vi "UHR-Fleezers Control (host) - 12.3.vi"() -> ()   [LabVIEW 2012] (continued)
                                }
                                frame #3 {
                                n359 = for {
                                N: 4 -> [_]
                                n360 = flat-sequence {
                                frame #0 {
                                n361 = Wait (ms)(milliseconds to wait=u32 500) -> ()  [unwired: 1 out]
                                }
                                frame #1 {
                                n362 = local read "Action (%)"() -> (w633:dbl)
                                n363 = Absolute Value(x=w633) -> (abs(x)=w632:dbl)
                                n364 = Greater?(x=w632, y=70.0) -> (0:w630:bool)
                                n365 = property on="Remove Action Offset" class="Bool (strict)"("Val(Sgnl)"=w630) -> ()  [unwired: 2 in, 2 out]
                                }
                                }
                                }
                                }
                                frame #4 {
                                n366 = Wait (ms)(milliseconds to wait=u32 500) -> ()  [unwired: 1 out]
                                }
                                frame #5 {
                                n367 = local read "Mean"() -> (w641:dbl)
                                n368 = Greater?(x=w641, y=11.0) -> (0:w635:bool)
                                n369 = Not(x=w635) -> (.not. x?=w636:bool)
                                n370 = And(x=w636, y="Shift confocal") -> (x .and. y?=w638:bool)
                                n371 = And(x=w635, y="Shift confocal") -> (x .and. y?=w639:bool)
                                n372 = case shown="True" w639 {
                                frame False {
                                }
                                frame True {
                                n373 = local read "Confocal Y 2 (V)"() -> (w645:dbl)
                                n374 = local read "Confocal X 2 (V)"() -> (w644:dbl)
                                n375 = property on="AO1" class="Slide (strict)"("Val(Sgnl)"=w645) -> ()  [unwired: 2 in, 2 out]
                                n376 = property on="AO2" class="Slide (strict)"("Val(Sgnl)"=w644) -> ()  [unwired: 2 in, 2 out]
                                }
                                }
                                n377 = case shown="True" w638 {
                                frame False {
                                }
                                frame True {
                                n378 = local read "Confocal Y 1 (V)"() -> (w643:dbl)
                                n379 = local read "Confocal X 1 (V)"() -> (w642:dbl)
                                n380 = property on="AO1" class="Slide (strict)"("Val(Sgnl)"=w643) -> ()  [unwired: 2 in, 2 out]
                                n381 = property on="AO2" class="Slide (strict)"("Val(Sgnl)"=w642) -> ()  [unwired: 2 in, 2 out]
                                }
                                }
                                }
                                frame #6 {
                                n382 = Wait (ms)(milliseconds to wait=u32 1500) -> ()  [unwired: 1 out]
                                }
                                frame #7 {
                                n383 = property on="Rem fb disp offset" class="Bool (strict)"("Val(Sgnl)"=TRUE ("Value (Signaling)")) -> ()  [unwired: 2 in, 2 out]
                                }
                                }
                                }
                                frame True {
                                n384 = flat-sequence {
                                tunnel: w648 -> [w649]
                                frame #0 {
                                n385 = property on="Trap Delta (MHz)" class="DigNum (strict)"("Val(Sgnl)"=w649) -> ()  [unwired: 2 in, 2 out]
                                }
                                frame #1 {
                                n386 = Wait (ms)(milliseconds to wait=u32 500) -> ()  [unwired: 1 out]
                                }
                                frame #2 {
                                n387 = local read "Shift confocal"() -> (w655:bool)
                                n388 = local read "Mean"() -> (w657:dbl)
                                n389 = Greater?(x=w657, y=11.0) -> (0:w654:bool)
                                n390 = Not(x=w654) -> (.not. x?=w653:bool)
                                n391 = And(x=w653, y=w655) -> (x .and. y?=w651:bool)
                                n392 = And(x=w654, y=w655) -> (x .and. y?=w652:bool)
                                n393 = case shown="True" w652 {
                                frame False {
                                }
                                frame True {
                                n394 = local read "Confocal Y 2 (V)"() -> (w661:dbl)
                                n395 = local read "Confocal X 2 (V)"() -> (w660:dbl)
                                n396 = property on="AO2" class="Slide (strict)"("Val(Sgnl)"=w660) -> ()  [unwired: 2 in, 2 out]
                                n397 = property on="AO1" class="Slide (strict)"("Val(Sgnl)"=w661) -> ()  [unwired: 2 in, 2 out]
                                }
                                }
                                n398 = case shown="True" w651 {
                                frame False {
                                }
                                frame True {
                                n399 = local read "Confocal X 1 (V)"() -> (w658:dbl)
                                n400 = local read "Confocal Y 1 (V)"() -> (w659:dbl)
                                n401 = property on="AO2" class="Slide (strict)"("Val(Sgnl)"=w658) -> ()  [unwired: 2 in, 2 out]
                                n402 = property on="AO1" class="Slide (strict)"("Val(Sgnl)"=w659) -> ()  [unwired: 2 in, 2 out]
                                }
                                }
                                }
                                }
                                }
                                }
                                }
                                }
                                }
                                frame "Image" {
                                n403 = property on="Confocal Image" class="Bool (strict)"("Val(Sgnl)"=TRUE ("Value (Signaling)")) -> ()  [unwired: 2 in, 2 out]
                                }
                              }
                              n404 = local write "Fl. High"(FALSE ("Fl. High")) -> ()
                              n405 = local read "Time (s)"() -> (w595:dbl)
                            }
                            frame #1 {
                              n406 = case shown="True" "Auto F Reset" {
                                tunnel: w667 -> [_ w672]
                                tunnel: w666 -> [_ w671]
                                tunnel: w665 -> [_ w670]
                                tunnel: w664 -> [_ w669]
                                frame False {
                                }
                                frame True {
                                n407 = node-c288() -> (w674:T21)  [unwired: 4 in]
                                n408 = timed-loop {
                                timing: w674 -> [_]
                                timing-out: [_] -> w673
                                tunnel: w672 -> [w679]
                                tunnel: w671 -> [w678]
                                tunnel: w670 -> [w677]
                                tunnel: w669 -> [w676]
                                stop <- w675 stop-if-true
                                n409 = node-c288() -> ()  [unwired: 1 in, 1 out]
                                n410 = local read "Fl. Delta Thresh. (kHz)"() -> (w688:dbl)
                                n411 = local read "APD to Watch"() -> (w689:bool)
                                n412 = local read "Delta Fl. 1"() -> (w690:dbl)
                                n413 = local read "Delta Fl. 2"() -> (w691:dbl)
                                n414 = local read "Fl. Triggered..."() -> (w682:bool)
                                n415 = local read "Stop All"() -> (w683:bool)
                                n416 = local read "Reset Force"() -> (w681:bool)
                                n417 = Multiply(x=w688, y=1000.0) -> (x*y=w686:dbl)
                                n418 = Select(t=w690, s=w689, f=w691) -> (s? t:f=w685:dbl)
                                n419 = Not(x=w682) -> (.not. x?=w680:bool)
                                n420 = Greater?(x=w685, y=w686) -> (0:w684:bool)
                                n421 = Compound Arithmetic op=OR(w684, w683, w680, w681) -> (w675:bool)
                                n422 = case shown="True" w675 {
                                tunnel: w679 -> [_ w695]
                                tunnel: w678 -> [_ w699]
                                tunnel: w677 -> [_ w698]
                                tunnel: w676 -> [_ w697]
                                frame False {
                                }
                                frame True {
                                n423 = case shown="\"Yank\"" w699 {
                                tunnel: w698 -> [_ w709]
                                tunnel: w697 -> [_ w707]
                                frame "Image", Default {
                                }
                                frame "Yank" {
                                n424 = flat-sequence {
                                tunnel: [w712] -> w710
                                tunnel: w709 -> [w712]
                                tunnel: [w711] -> w708
                                tunnel: w707 -> [w711]
                                tunnel: w710 -> [w718]
                                tunnel: w708 -> [w716]
                                frame #0 {
                                n425 = local read "Yank Delay (s)"() -> (w715:dbl)
                                n426 = Multiply(x=w715, y=1000.0) -> (x*y=w713:dbl)
                                n427 = Wait (ms)(milliseconds to wait=w713) -> ()  [unwired: 1 out]
                                }
                                frame #1 {
                                n428 = local read "Yank to which?"() -> (w717:bool)
                                n429 = case shown="False" w717 {
                                tunnel: w718 -> [_ w746]
                                tunnel: w716 -> [w719 _]
                                frame False {
                                n430 = flat-sequence {
                                tunnel: w719 -> [w720]
                                frame #0 {
                                n431 = property on="Trap Pos FB SP" class="DigNum (strict)"("Val(Sgnl)"=w720) -> ()  [unwired: 2 in, 2 out]
                                }
                                frame #1 {
                                n432 = Wait (ms)(milliseconds to wait=u32 700) -> ()  [unwired: 1 out]
                                }
                                frame #2 {
                                n433 = local read "Action (%)"() -> (w725:dbl)
                                n434 = Absolute Value(x=w725) -> (abs(x)=w724:dbl)
                                n435 = Greater?(x=w724, y=70.0) -> (0:w722:bool)
                                n436 = property on="Remove Action Offset" class="Bool (strict)"("Val(Sgnl)"=w722) -> ()  [unwired: 2 in, 2 out]
                                }
                                frame #3 {
                                n437 = for {
                                N: 4 -> [_]
                                n438 = flat-sequence {
                                frame #0 {
                                n439 = Wait (ms)(milliseconds to wait=u32 500) -> ()  [unwired: 1 out]
                                }
                                frame #1 {
                                n440 = local read "Action (%)"() -> (w731:dbl)
                                n441 = Absolute Value(x=w731) -> (abs(x)=w730:dbl)
                                n442 = Greater?(x=w730, y=70.0) -> (0:w728:bool)
                                n443 = property on="Remove Action Offset" class="Bool (strict)"("Val(Sgnl)"=w728) -> ()  [unwired: 2 in, 2 out]
                                }
                                }
                                }
                                }
                                frame #4 {
                                n444 = Wait (ms)(milliseconds to wait=u32 500) -> ()  [unwired: 1 out]
                                }
                                frame #5 {
                                n445 = local read "Shift confocal"() -> (w736:bool)
                                n446 = local read "Mean"() -> (w739:dbl)
                                n447 = Greater?(x=w739, y=11.0) -> (0:w735:bool)
                                n448 = Not(x=w735) -> (.not. x?=w734:bool)
                                n449 = And(x=w735, y=w736) -> (x .and. y?=w737:bool)
                                n450 = And(x=w734, y=w736) -> (x .and. y?=w733:bool)
                                n451 = case shown="True" w737 {
                                frame False {
                                }
                                frame True {
                                n452 = local read "Confocal X 2 (V)"() -> (w742:dbl)
                                n453 = local read "Confocal Y 2 (V)"() -> (w743:dbl)
                                n454 = property on="AO2" class="Slide (strict)"("Val(Sgnl)"=w742) -> ()  [unwired: 2 in, 2 out]
                                n455 = property on="AO1" class="Slide (strict)"("Val(Sgnl)"=w743) -> ()  [unwired: 2 in, 2 out]
                                }
                                }
                                n456 = case shown="True" w733 {
                                frame False {
                                }
                                frame True {
                                n457 = local read "Confocal Y 1 (V)"() -> (w741:dbl)
                                n458 = local read "Confocal X 1 (V)"() -> (w740:dbl)
                                n459 = property on="AO1" class="Slide (strict)"("Val(Sgnl)"=w741) -> ()  [unwired: 2 in, 2 out]
                                n460 = property on="AO2" class="Slide (strict)"("Val(Sgnl)"=w740) -> ()  [unwired: 2 in, 2 out]
                                }
                                }
                                }
                                frame #6 {
                                n461 = Wait (ms)(milliseconds to wait=u32 1500) -> ()  [unwired: 1 out]
                                }
                                frame #7 {
                                n462 = property on="Rem fb disp offset" class="Bool (strict)"("Val(Sgnl)"=TRUE ("Value (Signaling)")) -> ()  [unwired: 2 in, 2 out]
                                }
                                }
                                }
                                frame True {
                                n463 = flat-sequence {
                                tunnel: w746 -> [w747]
                                frame #0 {
                                n464 = property on="Trap Delta (MHz)" class="DigNum (strict)"("Val(Sgnl)"=w747) -> ()  [unwired: 2 in, 2 out]
                                }
                                frame #1 {
                                n465 = Wait (ms)(milliseconds to wait=u32 500) -> ()  [unwired: 1 out]
                                }
                                frame #2 {
                                n466 = local read "Shift confocal"() -> (w753:bool)
                                n467 = local read "Mean"() -> (w754:dbl)
                                n468 = Greater?(x=w754, y=11.0) -> (0:w752:bool)
                                n469 = And(x=w752, y=w753) -> (x .and. y?=w750:bool)
                                n470 = Not(x=w752) -> (.not. x?=w751:bool)
                                n471 = And(x=w751, y=w753) -> (x .and. y?=w749:bool)
                                n472 = case shown="True" w750 {
                                frame False {
                                }
                                frame True {
                                n473 = local read "Confocal Y 2 (V)"() -> (w759:dbl)
                                n474 = local read "Confocal X 2 (V)"() -> (w758:dbl)
                                n475 = property on="AO1" class="Slide (strict)"("Val(Sgnl)"=w759) -> ()  [unwired: 2 in, 2 out]
                                n476 = property on="AO2" class="Slide (strict)"("Val(Sgnl)"=w758) -> ()  [unwired: 2 in, 2 out]
                                }
                                }
                                n477 = case shown="True" w749 {
                                frame False {
                                }
                                frame True {
                                n478 = local read "Confocal Y 1 (V)"() -> (w757:dbl)
                                n479 = local read "Confocal X 1 (V)"() -> (w756:dbl)
                                n480 = property on="AO2" class="Slide (strict)"("Val(Sgnl)"=w756) -> ()  [unwired: 2 in, 2 out]
                                n481 = property on="AO1" class="Slide (strict)"("Val(Sgnl)"=w757) -> ()  [unwired: 2 in, 2 out]
                                }
                                }
                                }
                                }
                                }
                                }
                                }
                                }
                                }
                                }
                                n482 = local read "Time (s)"() -> (w694:dbl)
                                n483 = Subtract(x=w695, y=w694) -> (x-y=w706:dbl)
                                n484 = Number To Decimal String(number=w706, width (-)=i16 0) -> (decimal integer string=w704:string)
                                n485 = Concatenate Strings(w704, " s fluorescence event") -> (w701:string)
                                n486 = local read "Messages"() -> (w702:string)
                                n487 = local write "Duration (s)"(w706) -> ()
                                n488 = call "Update messages.vi"("Message to add"=w701, "Old message string"=w702) -> ("New message string"=w700:string)
                                n489 = local write "Messages"(w700) -> ()
                                n490 = call <vilib>:"Beep.vi"() -> ()  [unwired: 12 in]
                                n491 = local write "Reset Force"(FALSE ("Force Reset")) -> ()
                                n492 = local write "Fl. High"(TRUE ("Fl. High")) -> ()
                                n493 = local write "Waiting"(TRUE ("Waiting")) -> ()
                                }
                                }
                                n494 = node-c288() -> ()  [unwired: 1 in, 1 out]
                                }
                                n495 = node-c288(w673) -> ()  [unwired: 1 out]
                                }
                              }
                            }
                          }
                          n496 = local read "Trap Delta (MHz)"() -> (w585:dbl)
                          n497 = local read "Trap Pos FB SP"() -> (w583:fxp<+/-,16,1>)
                        }
                      }
                    }
                    frame True {
                      n498 = flat-sequence {
                        tunnel: w770 -> [w780]
                        tunnel: [w780] -> w774
                        tunnel: w773 -> [w779]
                        tunnel: [w779] -> w772
                        tunnel: [w778] -> w771
                        tunnel: w769 -> [w777]
                        tunnel: [w776] -> w768
                        tunnel: w765 -> [w775]
                        tunnel: [w775] -> w764
                        tunnel: w774 -> [w850]
                        tunnel: w772 -> [w849]
                        tunnel: w771 -> [w848]
                        tunnel: w768 -> [w847]
                        tunnel: w764 -> [w846]
                        tunnel: [w847] -> w767
                        frame #0 {
                          n499 = call <vilib>:"Beep.vi"() -> ()  [unwired: 3 in, 9 out]
                          n500 = local write "Waiting"(FALSE ("Waiting")) -> ()
                          n501 = Increment(x=w777) -> (x+1=w776:u8)
                          n502 = case shown="\"Yank\"" w779 {
                            tunnel: w776 -> [_ _ w786]
                            frame "Image" {
                              n503 = property on="Confocal Image" class="Bool (strict)"("Val(Sgnl)"=TRUE ("Value (Signaling)")) -> ()  [unwired: 2 in, 2 out]
                            }
                            frame "Alarm", Default {
                            }
                            frame "Yank" {
                              n504 = flat-sequence {
                                tunnel: w786 -> [w789]
                                tunnel: [w788] -> w785
                                tunnel: ["N Array El"] -> w784
                                tunnel: w785 -> [w803]
                                tunnel: w784 -> [w799]
                                frame #0 {
                                n505 = Multiply(x="Yank Delay (s)", y=1000.0) -> (x*y=w792:dbl)
                                n506 = Quotient & Remainder(x=w789, y="N Array El") -> (x-y*floor(x/y)=w788:u8)  [unwired: 1 out]
                                n507 = Wait (ms)(milliseconds to wait=w792) -> ()  [unwired: 1 out]
                                }
                                frame #1 {
                                n508 = Random Number (0-1)() -> (number: 0 to 1=w800:dbl)
                                n509 = Multiply(x=w799, y=w800) -> (x*y=w798:dbl)
                                n510 = Round Toward -Infinity(1:w798) -> (0:w797:dbl)
                                n511 = Select(t=w797, s="Random Choice", f=w803) -> (s? t:f=w801:dbl)
                                n512 = Select(t="Yank to Trap Delta (MHz)", s="Yank to which?", f="Yank to SP") -> (s? t:f=w794:dbl[])
                                n513 = Index Array(array=w794, index=w801) -> (element=w804:dbl)
                                n514 = case shown="False" "Yank to which?" {
                                tunnel: w804 -> [w805 w831]
                                frame False {
                                n515 = flat-sequence {
                                tunnel: w805 -> [w806]
                                frame #0 {
                                n516 = property on="Trap Pos FB SP" class="DigNum (strict)"("Val(Sgnl)"=w806) -> ()  [unwired: 2 in, 2 out]
                                }
                                frame #1 {
                                n517 = Wait (ms)(milliseconds to wait=u32 700) -> ()  [unwired: 1 out]
                                }
                                frame #2 {
                                n518 = local read "Action (%)"() -> (w811:dbl)
                                n519 = Absolute Value(x=w811) -> (abs(x)=w810:dbl)
                                n520 = Greater?(x=w810, y=70.0) -> (0:w808:bool)
                                n521 = property on="Remove Action Offset" class="Bool (strict)"("Val(Sgnl)"=w808) -> ()  [unwired: 2 in, 2 out]
                                }
                                frame #3 {
                                n522 = for {
                                N: 4 -> [_]
                                n523 = flat-sequence {
                                frame #0 {
                                n524 = Wait (ms)(milliseconds to wait=u32 500) -> ()  [unwired: 1 out]
                                }
                                frame #1 {
                                n525 = local read "Action (%)"() -> (w817:dbl)
                                n526 = Absolute Value(x=w817) -> (abs(x)=w816:dbl)
                                n527 = Greater?(x=w816, y=70.0) -> (0:w814:bool)
                                n528 = property on="Remove Action Offset" class="Bool (strict)"("Val(Sgnl)"=w814) -> ()  [unwired: 2 in, 2 out]
                                }
                                }
                                }
                                }
                                frame #4 {
                                n529 = local read "Shift confocal"() -> (w821:bool)
                                n530 = local read "Mean"() -> (w824:dbl)
                                n531 = Greater?(x=w824, y=11.0) -> (0:w820:bool)
                                n532 = Not(x=w820) -> (.not. x?=w819:bool)
                                n533 = And(x=w819, y=w821) -> (x .and. y?=w818:bool)
                                n534 = And(x=w820, y=w821) -> (x .and. y?=w822:bool)
                                n535 = case shown="True" w822 {
                                frame False {
                                }
                                frame True {
                                n536 = local read "Confocal X 2 (V)"() -> (w827:dbl)
                                n537 = local read "Confocal Y 2 (V)"() -> (w828:dbl)
                                n538 = property on="AO2" class="Slide (strict)"("Val(Sgnl)"=w827) -> ()  [unwired: 2 in, 2 out]
                                n539 = property on="AO1" class="Slide (strict)"("Val(Sgnl)"=w828) -> ()  [unwired: 2 in, 2 out]
                                }
                                }
                                n540 = case shown="True" w818 {
                                frame False {
                                }
                                frame True {
                                n541 = local read "Confocal X 1 (V)"() -> (w825:dbl)
                                n542 = local read "Confocal Y 1 (V)"() -> (w826:dbl)
                                n543 = property on="AO1" class="Slide (strict)"("Val(Sgnl)"=w826) -> ()  [unwired: 2 in, 2 out]
                                n544 = property on="AO2" class="Slide (strict)"("Val(Sgnl)"=w825) -> ()  [unwired: 2 in, 2 out]
                                }
                                }
                                }
                                frame #5 {
                                n545 = Wait (ms)(milliseconds to wait=u32 1500) -> ()  [unwired: 1 out]
                                }
                                frame #6 {
                                n546 = property on="Rem fb disp offset" class="Bool (strict)"("Val(Sgnl)"=TRUE ("Value (Signaling)")) -> ()  [unwired: 2 in, 2 out]
                                }
                                }
                                }
                                frame True {
                                n547 = flat-sequence {
                                tunnel: w831 -> [w832]
                                frame #0 {
                                n548 = property on="Trap Delta (MHz)" class="DigNum (strict)"("Val(Sgnl)"=w832) -> ()  [unwired: 2 in, 2 out]
                                }
                                frame #1 {
                                n549 = Wait (ms)(milliseconds to wait=u32 500) -> ()  [unwired: 1 out]
                                }
                                frame #2 {
                                n550 = local read "Shift confocal"() -> (w836:bool)
                                n551 = local read "Mean"() -> (w834:dbl)
                                n552 = Greater?(x=w834, y=11.0) -> (0:w837:bool)
                                n553 = Not(x=w837) -> (.not. x?=w838:bool)
                                n554 = And(x=w838, y=w836) -> (x .and. y?=w840:bool)
                                n555 = And(x=w837, y=w836) -> (x .and. y?=w839:bool)
                                n556 = case shown="True" w839 {
                                frame False {
                                }
                                frame True {
                                n557 = local read "Confocal Y 2 (V)"() -> (w844:dbl)
                                n558 = local read "Confocal X 2 (V)"() -> (w843:dbl)
                                n559 = property on="AO1" class="Slide (strict)"("Val(Sgnl)"=w844) -> ()  [unwired: 2 in, 2 out]
                                n560 = property on="AO2" class="Slide (strict)"("Val(Sgnl)"=w843) -> ()  [unwired: 2 in, 2 out]
                                }
                                }
                                n561 = case shown="True" w840 {
                                frame False {
                                }
                                frame True {
                                n562 = local read "Confocal X 1 (V)"() -> (w841:dbl)
                                n563 = local read "Confocal Y 1 (V)"() -> (w842:dbl)
                                n564 = property on="AO2" class="Slide (strict)"("Val(Sgnl)"=w841) -> ()  [unwired: 2 in, 2 out]
                                n565 = property on="AO1" class="Slide (strict)"("Val(Sgnl)"=w842) -> ()  [unwired: 2 in, 2 out]
                                }
                                }
                                }
                                }
                                }
                                }
                                }
                              }
                            }
                          }
                          n566 = local read "Time (s)"() -> (w778:dbl)
                          "Fl. High" <- TRUE ("Yanking")
                        }
                        frame #1 {
                          n567 = local read "Auto F Reset"() -> (w845:bool)
                          n568 = case shown="True" w845 {
                            tunnel: w850 -> [_ w854]
                            tunnel: w849 -> [_ w853]
                            tunnel: w848 -> [_ w852]
                            tunnel: w846 -> [_ w851]
                            frame False {
                            }
                            frame True {
                              n569 = node-c288() -> (w856:T21)  [unwired: 4 out]
                              n570 = timed-loop {
                                timing: w856 -> [_]
                                timing-out: [_] -> w855
                                tunnel: w854 -> [w874]
                                tunnel: w853 -> [w873]
                                tunnel: w852 -> [w872]
                                tunnel: w851 -> [w871]
                                stop <- w857 stop-if-true
                                n571 = node-c288() -> ()  [unwired: 2 out]
                                n572 = local read "Fl. Delta Thresh. (kHz)"() -> (w865:dbl)
                                n573 = local read "Fl. Triggered..."() -> (w870:bool)
                                n574 = local read "Delta Fl. 1"() -> (w861:dbl)
                                n575 = local read "Delta Fl. 2"() -> (w859:dbl)
                                n576 = local read "Stop All"() -> (w868:bool)
                                n577 = local read "APD to Watch"() -> (w860:bool)
                                n578 = Select(t=w861, s=w860, f=w859) -> (s? t:f=w858:dbl)
                                n579 = Not(x=w870) -> (.not. x?=w869:bool)
                                n580 = Multiply(x=w865, y=1000.0) -> (x*y=w864:dbl)
                                n581 = Negate(x=w864) -> (-x=w863:dbl)
                                n582 = Less?(x=w858, y=w863) -> (x < y?=w867:bool)
                                n583 = Compound Arithmetic op=OR(w867, w868, w869, "Reset Force") -> (w857:bool)
                                n584 = case shown="True" w857 {
                                tunnel: w874 -> [_ w889]
                                tunnel: w873 -> [_ w888]
                                tunnel: w872 -> [_ w878]
                                tunnel: w871 -> [_ w880]
                                frame False {
                                }
                                frame True {
                                n585 = local read "Time (s)"() -> (w879:dbl)
                                n586 = case shown="\"Yank\"" w888 {
                                tunnel: w889 -> [_ w892]
                                tunnel: w880 -> [_ w890]
                                frame "Image", Default {
                                }
                                frame "Yank" {
                                n587 = flat-sequence {
                                tunnel: [w898] -> w893
                                tunnel: w892 -> [w898]
                                tunnel: [w894] -> w891
                                tunnel: w890 -> [w894]
                                tunnel: w893 -> [w901]
                                tunnel: w891 -> [w899]
                                frame #0 {
                                n588 = local read "Yank Delay (s)"() -> (w897:dbl)
                                n589 = Multiply(x=w897, y=1000.0) -> (x*y=w895:dbl)
                                n590 = Wait (ms)(milliseconds to wait=w895) -> ()  [unwired: 1 out]
                                }
                                frame #1 {
                                n591 = local read "Yank to which?"() -> (w900:bool)
                                n592 = case shown="False" w900 {
                                tunnel: w901 -> [_ w928]
                                tunnel: w899 -> [w902 _]
                                frame False {
                                n593 = flat-sequence {
                                tunnel: w902 -> [w903]
                                frame #0 {
                                n594 = property on="Trap Pos FB SP" class="DigNum (strict)"("Val(Sgnl)"=w903) -> ()  [unwired: 2 in, 2 out]
                                }
                                frame #1 {
                                n595 = Wait (ms)(milliseconds to wait=u32 700) -> ()  [unwired: 1 out]
                                }
                                frame #2 {
                                n596 = local read "Action (%)"() -> (w908:dbl)
                                n597 = Absolute Value(x=w908) -> (abs(x)=w907:dbl)
                                n598 = Greater?(x=w907, y=70.0) -> (0:w905:bool)
                                n599 = property on="Remove Action Offset" class="Bool (strict)"("Val(Sgnl)"=w905) -> ()  [unwired: 2 in, 2 out]
                                }
                                frame #3 {
                                n600 = for {
                                N: 4 -> [_]
                                n601 = flat-sequence {
                                frame #0 {
                                n602 = Wait (ms)(milliseconds to wait=u32 500) -> ()  [unwired: 1 out]
                                }
                                frame #1 {
                                n603 = local read "Action (%)"() -> (w914:dbl)
                                n604 = Absolute Value(x=w914) -> (abs(x)=w913:dbl)
                                n605 = Greater?(x=w913, y=70.0) -> (0:w911:bool)
                                n606 = property on="Remove Action Offset" class="Bool (strict)"("Val(Sgnl)"=w911) -> ()  [unwired: 2 in, 2 out]
                                }
                                }
                                }
                                }
                                frame #4 {
                                n607 = local read "Shift confocal"() -> (w919:bool)
                                n608 = local read "Mean"() -> (w921:dbl)
                                n609 = Greater?(x=w921, y=11.0) -> (0:w918:bool)
                                n610 = Not(x=w918) -> (.not. x?=w917:bool)
                                n611 = And(x=w918, y=w919) -> (x .and. y?=w916:bool)
                                n612 = And(x=w917, y=w919) -> (x .and. y?=w915:bool)
                                n613 = case shown="True" w916 {
                                frame False {
                                }
                                frame True {
                                n614 = local read "Confocal Y 2 (V)"() -> (w925:dbl)
                                n615 = local read "Confocal X 2 (V)"() -> (w924:dbl)
                                n616 = property on="AO2" class="Slide (strict)"("Val(Sgnl)"=w924) -> ()  [unwired: 2 in, 2 out]
                                n617 = property on="AO1" class="Slide (strict)"("Val(Sgnl)"=w925) -> ()  [unwired: 2 in, 2 out]
                                }
                                }
                                n618 = case shown="True" w915 {
                                frame False {
                                }
                                frame True {
                                n619 = local read "Confocal X 1 (V)"() -> (w922:dbl)
                                n620 = local read "Confocal Y 1 (V)"() -> (w923:dbl)
                                n621 = property on="AO1" class="Slide (strict)"("Val(Sgnl)"=w923) -> ()  [unwired: 2 in, 2 out]
                                n622 = property on="AO2" class="Slide (strict)"("Val(Sgnl)"=w922) -> ()  [unwired: 2 in, 2 out]
                                }
                                }
                                }
                                frame #5 {
                                n623 = Wait (ms)(milliseconds to wait=u32 1500) -> ()  [unwired: 1 out]
                                }
                                frame #6 {
                                n624 = property on="Rem fb disp offset" class="Bool (strict)"("Val(Sgnl)"=TRUE ("Value (Signaling)")) -> ()  [unwired: 2 in, 2 out]
                                }
                                }
                                }
                                frame True {
                                n625 = flat-sequence {
                                tunnel: w928 -> [w929]
                                frame #0 {
                                n626 = property on="Trap Delta (MHz)" class="DigNum (strict)"("Val(Sgnl)"=w929) -> ()  [unwired: 2 in, 2 out]
                                }
                                frame #1 {
                                n627 = Wait (ms)(milliseconds to wait=u32 500) -> ()  [unwired: 1 out]
                                }
                                frame #2 {
                                n628 = local read "Shift confocal"() -> (w935:bool)
                                n629 = local read "Mean"() -> (w937:dbl)
                                n630 = Greater?(x=w937, y=11.0) -> (0:w934:bool)
                                n631 = Not(x=w934) -> (.not. x?=w933:bool)
                                n632 = And(x=w934, y=w935) -> (x .and. y?=w932:bool)
                                n633 = And(x=w933, y=w935) -> (x .and. y?=w931:bool)
                                n634 = case shown="True" w932 {
                                frame False {
                                }
                                frame True {
                                n635 = local read "Confocal Y 2 (V)"() -> (w941:dbl)
                                n636 = local read "Confocal X 2 (V)"() -> (w940:dbl)
                                n637 = property on="AO2" class="Slide (strict)"("Val(Sgnl)"=w940) -> ()  [unwired: 2 in, 2 out]
                                n638 = property on="AO1" class="Slide (strict)"("Val(Sgnl)"=w941) -> ()  [unwired: 2 in, 2 out]
                                }
                                }
                                n639 = case shown="True" w931 {
                                frame False {
                                }
                                frame True {
                                n640 = local read "Confocal Y 1 (V)"() -> (w939:dbl)
                                n641 = local read "Confocal X 1 (V)"() -> (w938:dbl)
                                n642 = property on="AO2" class="Slide (strict)"("Val(Sgnl)"=w938) -> ()  [unwired: 2 in, 2 out]
                                n643 = property on="AO1" class="Slide (strict)"("Val(Sgnl)"=w939) -> ()  [unwired: 2 in, 2 out]
                                }
                                }
                                }
                                }
                                }
                                }
                                }
                                }
                                }
                                }
                                n644 = local read "Messages"() -> (w887:string)
                                n645 = Subtract(x=w879, y=w878) -> (x-y=w885:dbl)
                                "Duration (s)" <- w885
                                n646 = Number To Decimal String(number=w885, width (-)=i16 0) -> (decimal integer string=w883:string)
                                n647 = Concatenate Strings(w883, " s fluorescence event." ("string")) -> (w881:string)
                                n648 = call "Update messages.vi"("Message to add"=w881, "Old message string"=w887) -> ("New message string"=w886:string)
                                n649 = local write "Reset Force"(FALSE ("Reset Force")) -> ()
                                n650 = local write "Waiting"(TRUE ("Waiting")) -> ()
                                n651 = local write "Messages"(w886) -> ()
                                n652 = local write "Fl. High"(FALSE ("Fl. High")) -> ()
                                n653 = call <vilib>:"Beep.vi"() -> ()  [unwired: 3 in, 9 out]
                                }
                                }
                                n654 = node-c288() -> ()  [unwired: 2 out]
                              }
                              n655 = node-c288(w855) -> ()  [unwired: 1 out]
                            }
                          }
                        }
                      }
                      n656 = local read "Trap Delta (MHz)"() -> (w770:dbl)
                      n657 = local read "Trap Pos FB SP"() -> (w765:fxp<+/-,16,1>)
                    }
                  }
                }
                frame #1 {
                  n658 = local read "Stop All"() -> (w951:bool)
                  n659 = local read "Fl. Triggered..."() -> (w949:bool)
                  n660 = Not(x=w949) -> (.not. x?=w950:bool)
                  n661 = Or(x=w950, y=w951) -> (x .or. y?=w948:bool)
                }
              }
              n662 = case shown="True" w542 {
                frame False {
                }
                frame True {
                  n663 = local read "Confocal Y 1 (V)"() -> (w552:dbl)
                  n664 = local read "Confocal X 1 (V)"() -> (w551:dbl)
                  n665 = property on="AO2" class="Slide (strict)"("Val(Sgnl)"=w551) -> ()  [unwired: 2 in, 2 out]
                  n666 = property on="AO1" class="Slide (strict)"("Val(Sgnl)"=w552) -> ()  [unwired: 2 in, 2 out]
                }
              }
              n667 = case shown="True" w542 {
                frame False {
                }
                frame True {
                  w550 = FALSE ("Fl. High")
                  n668 = local write "Waiting"(w550) -> ()
                  n669 = local write "Fl. High"(w550) -> ()
                }
              }
              n670 = node-c288() -> ()  [unwired: 2 out]
            }
            n671 = node-c288(w540) -> ()  [unwired: 1 out]
          }
        }
      }
      event "Stop All": Value Change {
        n672 = event-data() -> ()  [unwired: 7 out]
        n673 = local read "Stop All"() -> (w956:bool)
      }
    }
    n674 = node-c288() -> ()  [unwired: 2 out]
  }
  n675 = timed-loop "Run Scripts, including: stage motion" {
    tunnel: w114 -> [w963]
    tunnel: w113 -> [w964]
    tunnel: [w964] -> w112
    tunnel: [w963] -> w111
    timing: w109 -> [_]
    timing-out: [_] -> w108
    tunnel: w95 -> [w962]
    tunnel: w96 -> [w961]
    tunnel: w67 -> [w958]
    tunnel: w66 -> [w957]
    tunnel: w65 -> [w959]
    tunnel: w64 -> [w960]
    stop <- w965 stop-if-true
    n676 = node-c288() -> ()  [unwired: 1 in, 1 out]
    n677 = event shown="[7] \"Dump Beads\": Value Change" {
      selector: _ -> [_ _ _ _ _ _ _ _ _ _ _ _ _ _ _ _ _ _ _]
      dyn-events: _ -> [_ _ _ _ _ _ _ _ _ _ _ _ _ _ _ _ _ _ _]
      timeout: _ -> [_ _ _ _ _ _ _ _ _ _ _ _ _ _ _ _ _ _ _]
      tunnel: ["Set Position" "Move to Position" _ _ "Read Harvard" _ _ _ _ _ _ "Got ADig bead" "Force FB Data\nScript" _ "Got DNA bead" "Take Stepping Data" _ "Take Detection Laser\nImage" _] -> _
      tunnel: [_ _ _ _ _ _ _ _ _ _ _ _ _ _ _ _ _ _ w1582] -> w965
      tunnel: w963 -> [w983 w991 w1004 w1034 _ w1079 w1119 w1200 w1229 w1361 w1387 _ w1423 _ _ _ _ _ _]
      tunnel: w964 -> [w984 w992 w1005 w1035 _ w1080 w1120 w1201 w1230 w1362 w1388 _ w1424 _ _ _ _ _ _]
      tunnel: w962 -> [_ _ _ _ w1064 _ _ _ _ _ _ _ _ _ _ _ _ _ _]
      tunnel: w961 -> [_ _ _ _ w1063 _ _ _ _ _ _ _ _ _ _ _ _ _ _]
      tunnel: w960 -> [_ _ _ _ _ _ _ _ _ _ _ _ _ _ _ _ _ _ _]
      tunnel: w959 -> [_ _ _ _ _ _ _ _ _ _ _ _ _ _ _ _ _ _ _]
      tunnel: w958 -> [_ _ _ _ _ _ _ _ _ _ _ _ _ _ _ _ _ _ _]
      tunnel: w957 -> [_ _ _ _ _ _ _ _ _ _ _ _ _ _ _ _ _ _ _]
      event "Set Position", "Set Position 2", "Set Position 3", "Set Position 4", "Set Position 5", "Set Position 1": Value Change {
        n678 = event-data() -> ()  [unwired: 1 in, 5 out]
        n679 = Build Array("Set Position 1", "Set Position 2", "Set Position 3", "Set Position 4", "Set Position 5") -> (w982:bool[])
        n680 = Boolean Array To Number(Boolean array=w982) -> (number=w981:u32)
        n681 = Logarithm Base 2(1:w981) -> (0:w973:dbl)
        n682 = call "Read Stage Position.vi"("error in"=w983, "VISA resource name in"=w984) -> ("Current Position"=w988:cluster{dbl, dbl, dbl}, "error out"=w987:errorcluster)  [unwired: 2 out]
        n683 = Decrement(x="Position") -> (x-1=w971:dbl)
        n684 = Greater Or Equal?(x=w973, y=0.0) -> (x >= y?=w974:bool)
        n685 = Cluster To Array(cluster=w988) -> (array=w985:dbl[])
        n686 = local write "Stage Control Serial Error"(w987) -> ()
        n687 = Select(t=w973, s=w974, f=w971) -> (s? t:f=w970:dbl)
        n688 = Increment(x=w970) -> (x+1=w969:dbl)
        n689 = Build Array (concatenate)(w969, w985) -> (w968:dbl[])
        n690 = Replace Array Subset(array="Saved Stage Positions", new element=w968, index (row)=w970) -> (w986:dbl[][])  [unwired: 1 in]
        n691 = local write "Saved Stage Positions"(w986) -> ()
      }
      event "Move to Position": Value Change {
        n692 = event-data() -> ()  [unwired: 1 in, 5 out]
        n693 = flat-sequence {
          tunnel: w992 -> [w996]
          tunnel: w991 -> [w995]
          frame #0 {
            n694 = local read "Saved Stage Positions"() -> (w998:dbl[][])
            n695 = local read "Position"() -> (w997:dbl)
            n696 = local write "Stage Moving"(TRUE ("Stage Moving")) -> ()
            n697 = call "move to saved stage position.vi"("error in"=w995, "Stage VISA resource name in"=w996, "Position"=w997, "Saved Stage Positions"=w998) -> ("error out"=w994:errorcluster)  [unwired: 1 out]
            n698 = local write "Stage Control Serial Error"(w994) -> ()
          }
          frame #1 {
            n699 = call <vilib>:"Beep.vi"() -> ()  [unwired: 3 in, 9 out]
            n700 = local write "Stage Moving"(FALSE ("Stage Moving")) -> ()
          }
        }
      }
      event "Move Cap. 1 (DNA Bottom)": Value Change {
        n701 = event-data() -> ()  [unwired: 1 in, 5 out]
        n702 = local write "Move Cap. 1 (DNA Bottom)"(FALSE ("Move Cap. 1 (DNA Right)")) -> ()
        n703 = flat-sequence {
          tunnel: w1004 -> [w1007]
          tunnel: w1005 -> [w1008]
          tunnel: [w1008] -> w1002
          tunnel: [w1007] -> w1001
          tunnel: w1002 -> [w1010]
          tunnel: w1001 -> [w1009]
          frame #0 {
            n704 = property on="Sample Channel\nFlow" class="Bool (strict)"("Val(Sgnl)"="Cap 1 Samp Flow ON") -> ()  [unwired: 2 in, 2 out]
          }
          frame #1 {
            n705 = local read "Saved Stage Positions"() -> (w1020:dbl[][])
            n706 = local write "Stage Moving"(TRUE ("Stage Moving")) -> ()
            n707 = Array Subset(array=w1020, index (row)=0 ("index"), length (row)=1 ("length"), index (col)=1 ("index"), length (col)=3 ("length")) -> (w1017:dbl[][])
            n708 = Reshape Array(w1017, 3 ("dimension size")) -> (w1015:dbl[])
            n709 = Array To Cluster(array=w1015) -> (cluster=w1014:cluster{"[0]":dbl, "[1]":dbl, "[2]":dbl})
            n710 = call "Set Stage Position.vi"("Position"=w1014, "error in"=w1009, "VISA resource name in"=w1010) -> ("error out"=w1013:errorcluster)  [unwired: 2 out]
            n711 = local write "Stage Control Serial Error"(w1013) -> ()
          }
          frame #2 {
            n712 = local write "Stage Moving"(FALSE ("Stage Moving")) -> ()
            n713 = case shown="True" "Cap 1 Flow ON" {
              frame False {
              }
              frame True {
                n714 = property on="Inject Pump 1" class="Bool (strict)"("Val(Sgnl)"=TRUE ("Value (Signaling)")) -> ()  [unwired: 2 in, 2 out]
              }
            }
            n715 = call <vilib>:"Beep.vi"() -> ()  [unwired: 3 in, 9 out]
          }
          frame #3 {
            n716 = property on="Sample Channel\nFlow" class="Bool (strict)"("Val(Sgnl)"=FALSE ("Value (Signaling)")) -> ()  [unwired: 2 in, 2 out]
            n717 = local read "Cap. 2 BD T1?\n(ADig T1, DNA T2)"() -> (w1027:bool)
            n718 = case shown="True" w1027 {
              tunnel: "Cap 1 T ON" -> [w1029 w1030]
              frame False {
                n719 = property on="Trap 1 (ON/OFF)" class="Bool (strict)"("Val(Sgnl)"=w1029) -> ()  [unwired: 2 in, 2 out]
              }
              frame True {
                n720 = property on="Trap 2 (ON/OFF)" class="Bool (strict)"("Val(Sgnl)"=w1030) -> ()  [unwired: 2 in, 2 out]
              }
            }
            n721 = property on="Got DNA bead" class="Bool"("Key Focus"=TRUE) -> ()  [unwired: 2 in, 2 out]
          }
        }
      }
      event "Move Cap. 2 (ADig Top)": Value Change {
        n722 = event-data() -> ()  [unwired: 1 in, 5 out]
        n723 = local write "Move Cap. 2 (ADig Top)"(FALSE ("Move Cap. 2 (ADig Left)")) -> ()
        n724 = flat-sequence {
          tunnel: w1034 -> [w1037]
          tunnel: w1035 -> [w1038]
          tunnel: [w1038] -> w1032
          tunnel: [w1037] -> w1031
          tunnel: w1032 -> [w1041]
          tunnel: w1031 -> [w1040]
          frame #0 {
            n725 = property on="Sample Channel\nFlow" class="Bool (strict)"("Val(Sgnl)"="Cap 2 Samp Flow ON") -> ()  [unwired: 2 in, 2 out]
          }
          frame #1 {
            w1039 = FALSE ("Value (Signaling)")
            n726 = local read "Saved Stage Positions"() -> (w1051:dbl[][])
            n727 = local write "Stage Moving"(TRUE ("Stage Moving")) -> ()
            n728 = Array Subset(array=w1051, index (row)=1 ("index"), length (row)=1 ("length"), index (col)=1 ("index"), length (col)=3 ("length")) -> (w1048:dbl[][])
            n729 = Reshape Array(w1048, 3 ("dimension size")) -> (w1046:dbl[])
            n730 = property on="Trap 1 (ON/OFF)" class="Bool (strict)"("Val(Sgnl)"=w1039) -> ()  [unwired: 2 in, 2 out]
            n731 = property on="Trap 1 (ON/OFF)" class="Bool (strict)"("Val(Sgnl)"=w1039) -> ()  [unwired: 2 in, 2 out]
            n732 = Array To Cluster(array=w1046) -> (cluster=w1045:cluster{"[0]":dbl, "[1]":dbl, "[2]":dbl})
            n733 = call "Set Stage Position.vi"("Position"=w1045, "error in"=w1040, "VISA resource name in"=w1041) -> ("error out"=w1044:errorcluster)  [unwired: 2 out]
            n734 = local write "Stage Control Serial Error"(w1044) -> ()
          }
          frame #2 {
            n735 = local write "Stage Moving"(FALSE ("Stage Moving")) -> ()
            n736 = call <vilib>:"Beep.vi"() -> ()  [unwired: 3 in, 9 out]
            n737 = case shown="True" "Cap 2 Flow ON" {
              frame False {
              }
              frame True {
                n738 = property on="Inject Pump 3" class="Bool (strict)"("Val(Sgnl)"=TRUE ("Value (Signaling)")) -> ()  [unwired: 2 in, 2 out]